vi "FlexMag - 23-03-2023.vi"() -> ()   [LabVIEW 2018] (continued)
        n7498 = feedback #256() -> (w13354:dbl)  [unwired: 1 in]
        n7499 = feedback-in #256(w13355) -> ()
        n7500 = feedback #257() -> (w13344:dbl)  [unwired: 1 in]
        n7501 = feedback-in #257(w13345) -> ()
        n7502 = feedback #258() -> (w13331:dbl)  [unwired: 1 in]
        n7503 = feedback-in #258(w13330) -> ()
        n7504 = feedback #259() -> (w13301:dbl)  [unwired: 1 in]
        n7505 = feedback-in #259(w13302) -> ()
        n7506 = feedback #260() -> (w13291:dbl)  [unwired: 1 in]
        n7507 = feedback-in #260(w13292) -> ()
        n7508 = feedback #261() -> (w13280:dbl)  [unwired: 1 in]
        n7509 = feedback-in #261(w13279) -> ()
        n7510 = feedback #262() -> (w13353:dbl)  [unwired: 1 in]
        n7511 = feedback-in #262(w13354) -> ()
        n7512 = feedback #263() -> (w13343:dbl)  [unwired: 1 in]
        n7513 = feedback-in #263(w13344) -> ()
        n7514 = feedback #264() -> (w13332:dbl)  [unwired: 1 in]
        n7515 = feedback-in #264(w13331) -> ()
        n7516 = feedback #265() -> (w13300:dbl)  [unwired: 1 in]
        n7517 = feedback-in #265(w13301) -> ()
        n7518 = feedback #266() -> (w13290:dbl)  [unwired: 1 in]
        n7519 = feedback-in #266(w13291) -> ()
        n7520 = feedback #267() -> (w13281:dbl)  [unwired: 1 in]
        n7521 = feedback-in #267(w13280) -> ()
        n7522 = feedback #268() -> (w13352:dbl)  [unwired: 1 in]
        n7523 = feedback-in #268(w13353) -> ()
        n7524 = feedback #269() -> (w13342:dbl)  [unwired: 1 in]
        n7525 = feedback-in #269(w13343) -> ()
        n7526 = feedback #270() -> (w13333:dbl)  [unwired: 1 in]
        n7527 = feedback-in #270(w13332) -> ()
        n7528 = feedback #271() -> (w13299:dbl)  [unwired: 1 in]
        n7529 = feedback-in #271(w13300) -> ()
        n7530 = feedback #272() -> (w13289:dbl)  [unwired: 1 in]
        n7531 = feedback-in #272(w13290) -> ()
        n7532 = feedback #273() -> (w13282:dbl)  [unwired: 1 in]
        n7533 = feedback-in #273(w13281) -> ()
        n7534 = feedback #274() -> (w13351:dbl)  [unwired: 1 in]
        n7535 = feedback-in #274(w13352) -> ()
        n7536 = feedback #275() -> (w13341:dbl)  [unwired: 1 in]
        n7537 = feedback-in #275(w13342) -> ()
        n7538 = feedback #276() -> (w13334:dbl)  [unwired: 1 in]
        n7539 = feedback-in #276(w13333) -> ()
        n7540 = feedback #277() -> (w13298:dbl)  [unwired: 1 in]
        n7541 = feedback-in #277(w13299) -> ()
        n7542 = feedback #278() -> (w13288:dbl)  [unwired: 1 in]
        n7543 = feedback-in #278(w13289) -> ()
        n7544 = feedback #279() -> (w13283:dbl)  [unwired: 1 in]
        n7545 = feedback-in #279(w13282) -> ()
        n7546 = feedback #280() -> (w13350:dbl)  [unwired: 1 in]
        n7547 = feedback-in #280(w13351) -> ()
        n7548 = feedback #281() -> (w13340:dbl)  [unwired: 1 in]
        n7549 = feedback-in #281(w13341) -> ()
        n7550 = feedback #282() -> (w13335:dbl)  [unwired: 1 in]
        n7551 = feedback-in #282(w13334) -> ()
        n7552 = feedback #283() -> (w13297:dbl)  [unwired: 1 in]
        n7553 = feedback-in #283(w13298) -> ()
        n7554 = feedback #284() -> (w13287:dbl)  [unwired: 1 in]
        n7555 = feedback-in #284(w13288) -> ()
        n7556 = feedback #285() -> (w13284:dbl)  [unwired: 1 in]
        n7557 = feedback-in #285(w13283) -> ()
        n7558 = feedback #286() -> (w13349:dbl)  [unwired: 1 in]
        n7559 = feedback-in #286(w13350) -> ()
        n7560 = feedback #287() -> (w13339:dbl)  [unwired: 1 in]
        n7561 = feedback-in #287(w13340) -> ()
        n7562 = feedback #288() -> (w13336:dbl)  [unwired: 1 in]
        n7563 = feedback-in #288(w13335) -> ()
        n7564 = feedback #289() -> (w13296:dbl)  [unwired: 1 in]
        n7565 = feedback-in #289(w13297) -> ()
        n7566 = feedback #290() -> (w13286:dbl)  [unwired: 1 in]
        n7567 = feedback-in #290(w13287) -> ()
        n7568 = feedback #291() -> (w13285:dbl)  [unwired: 1 in]
        n7569 = feedback-in #291(w13284) -> ()
        n7570 = feedback #292() -> (w13348:dbl)  [unwired: 1 in]
        n7571 = feedback-in #292(w13349) -> ()
        n7572 = feedback #293() -> (w13338:dbl)  [unwired: 1 in]
        n7573 = feedback-in #293(w13339) -> ()
        n7574 = feedback #294() -> (w13337:dbl)  [unwired: 1 in]
        n7575 = feedback-in #294(w13336) -> ()
        n7576 = Compound Arithmetic op=ADD(w13305, w13304, w13303, w13302, w13301, w13300, w13299, w13298, w13297, w13296) -> (w13308:dbl)
        n7577 = Compound Arithmetic op=ADD(w13295, w13294, w13293, w13292, w13291, w13290, w13289, w13288, w13287, w13286) -> (w13307:dbl)
        n7578 = Compound Arithmetic op=ADD(w13276, w13277, w13278, w13279, w13280, w13281, w13282, w13283, w13284, w13285) -> (w13306:dbl)
        n7579 = Compound Arithmetic op=ADD(w13357, w13356, w13355, w13354, w13353, w13352, w13351, w13350, w13349, w13348) -> (w13360:dbl)
        n7580 = Compound Arithmetic op=ADD(w13347, w13346, w13345, w13344, w13343, w13342, w13341, w13340, w13339, w13338) -> (w13359:dbl)
        n7581 = Compound Arithmetic op=ADD(w13328, w13329, w13330, w13331, w13332, w13333, w13334, w13335, w13336, w13337) -> (w13358:dbl)
        n7582 = Divide(x=w13308, y=10.0) -> (x/y=w13271:dbl)
        "ch4 cc ai(V)" <- w13271
        n7583 = Divide(x=w13360, y=10.0) -> (x/y=w13364:dbl)
        "ch3 cc ai(V)" <- w13364
        n7584 = Divide(x=w13307, y=10.0) -> (x/y=w13269:dbl)
        "ch4 pl pg ai(V)" <- w13269
        n7585 = Divide(x=w13306, y=10.0) -> (x/y=w13270:dbl)
        "ch4 ch pg ai(V)" <- w13270
        n7586 = Divide(x=w13359, y=10.0) -> (x/y=w13372:dbl)
        "ch3 pl pg ai(V)" <- w13372
        n7587 = Divide(x=w13358, y=10.0) -> (x/y=w13368:dbl)
        "ch3 ch pg ai(V)" <- w13368
        n7588 = Subtract(x=w13269, y=5.625) -> (x-y=w13268:dbl)
        n7589 = Subtract(x=w13270, y=5.625) -> (x-y=w13267:dbl)
        n7590 = Subtract(x=w13271, y=10.625) -> (x-y=w13261:dbl)
        n7591 = Subtract(x=w13372, y=5.625) -> (x-y=w13370:dbl)
        n7592 = Power Of 10(x=w13268) -> (10^x=w13266:dbl)
        n7593 = Subtract(x=w13368, y=5.625) -> (x-y=w13366:dbl)
        n7594 = Subtract(x=w13364, y=10.625) -> (x-y=w13362:dbl)
        n7595 = Power Of 10(x=w13261) -> (10^x=w13262:dbl)
        n7596 = Power Of 10(x=w13267) -> (10^x=w13264:dbl)
        n7597 = Power Of 10(x=w13370) -> (10^x=w13371:dbl)
        n7598 = Power Of 10(x=w13366) -> (10^x=w13365:dbl)
        n7599 = Power Of 10(x=w13362) -> (10^x=w13363:dbl)
        n7600 = In Range and Coerce(upper limit=1.0, x=w13262, lower limit=1e-09) -> (coerced(x)=w13260:dbl)  [unwired: 1 out]
        "ch4 cc torr" <- w13260
        n7601 = In Range and Coerce(upper limit=760.0, x=w13266, lower limit=0.000375) -> (coerced(x)=w13265:dbl)  [unwired: 1 out]
        "ch4 pl pg torr" <- w13265
        n7602 = In Range and Coerce(upper limit=760.0, x=w13371, lower limit=0.000375) -> (coerced(x)=w13369:dbl)  [unwired: 1 out]
        "ch3 pl pg  torr" <- w13369
        n7603 = In Range and Coerce(upper limit=760.0, x=w13264, lower limit=0.000375) -> (coerced(x)=w13263:dbl)  [unwired: 1 out]
        "ch4 ch pg torr" <- w13263
        n7604 = In Range and Coerce(upper limit=760.0, x=w13365, lower limit=0.000375) -> (coerced(x)=w13367:dbl)  [unwired: 1 out]
        "ch3 ch pg torr" <- w13367
        n7605 = In Range and Coerce(upper limit=1.0, x=w13363, lower limit=1e-09) -> (coerced(x)=w13361:dbl)  [unwired: 1 out]
        "ch3 cc torr" <- w13361
        n7606 = Multiply(x=w13260, y=1.33) -> (x*y=w13227:dbl)
        "ch4 cc mbar" <- w13227
        "ch4 cc mbar gui" <- w13227
        "ch4 cc mbar gui 1" <- w13227
        n7607 = Multiply(x=w13265, y=1.33) -> (x*y=w13229:dbl)
        "ch4 pl pg mbar" <- w13229
        "ch4 pl pg mbar gui" <- w13229
        "ch4 pl pg mbar gui 1" <- w13229
        n7608 = Multiply(x=w13369, y=1.33) -> (x*y=w13232:dbl)
        "ch3 pl pg mbar" <- w13232
        "ch3 pl pg mbar gui" <- w13232
        "ch3 pl pg mbar gui 1" <- w13232
        n7609 = Multiply(x=w13367, y=1.33) -> (x*y=w13231:dbl)
        "ch3 ch pg mbar" <- w13231
        "ch3 ch pg mbar gui" <- w13231
        "ch3 ch pg mbar gui 1" <- w13231
        n7610 = Multiply(x=w13361, y=1.33) -> (x*y=w13230:dbl)
        "ch3 cc mbar" <- w13230
        "ch3 cc mbar gui" <- w13230
        "ch3 cc mbar gui 1" <- w13230
        n7611 = Multiply(x=w13263, y=1.33) -> (x*y=w13228:dbl)
        "ch4 ch pg mbar" <- w13228
        "ch4 ch pg mbar gui" <- w13228
        "ch4 ch pg mbar gui 1" <- w13228
        n7612 = Number To Exponential String(number=w13231, precision (6)=i16 3) -> (E-format string=→"CH3 CH PG":string)  [unwired: 2 in]
        n7613 = Number To Exponential String(number=w13230, precision (6)=i16 3) -> (E-format string=→"CH3 CH CC":string)  [unwired: 2 in]
        n7614 = Number To Exponential String(number=w13232, precision (6)=i16 3) -> (E-format string=→"CH3 PL PG":string)  [unwired: 2 in]
        n7615 = Number To Exponential String(number=w13228, precision (6)=i16 3) -> (E-format string=→"CH4 CH PG":string)  [unwired: 2 in]
        n7616 = Number To Exponential String(number=w13227, precision (6)=i16 3) -> (E-format string=→"CH4 CH CC":string)  [unwired: 2 in]
        n7617 = Number To Exponential String(number=w13229, precision (6)=i16 3) -> (E-format string=→"CH4 PL PG":string)  [unwired: 2 in]
      }
    }
    n7618 = local read "MFC_Ar_Read_value"() -> (w12961:u16)
    n7619 = Wait Until Next ms Multiple(millisecond multiple=u32 300) -> ()  [unwired: 1 out]
    n7620 = Compound Arithmetic op=OR("ch1 ar set zero", "ch1 ar set zero auto") -> (w12986:bool)
    n7621 = Compound Arithmetic op=OR("ch4 ar set", "ch4 ar set auto") -> (w12990:bool)
    n7622 = Compound Arithmetic op=OR("ch4 ar set zero", "ch4 ar set zero auto") -> (w12989:bool)
    n7623 = Compound Arithmetic op=OR("ch1 ar set", "ch1 ar set auto") -> (w12983:bool)
    n7624 = Compound Arithmetic op=OR("ch2 ar set", "ch2 ar set auto") -> (w12994:bool)
    n7625 = Compound Arithmetic op=OR("ch2 ar set zero", "ch2 ar set zero auto") -> (w12995:bool)
    n7626 = Compound Arithmetic op=OR("ch3 ar set", "ch3 ar set auto") -> (w12997:bool)
    n7627 = Compound Arithmetic op=OR("ch3 ar set zero", "ch3 ar set zero auto") -> (w13005:bool)
    n7628 = Build Array(FALSE ("element"), w12983, w12986, w12994, w12995, w12997, w13005, w12990, w12989) -> (w12999:bool[])
    n7629 = Boolean Array To Number(Boolean array=w12999) -> (number=w13000:u32)
    n7630 = Less?(x=w12961, y=u16 20) -> (x < y?=w12964:bool)
    n7631 = Mantissa & Exponent(0:w13000) -> (2:w12998:dbl)  [unwired: 1 out]
    n7632 = case shown="False" w12964 {
      tunnel: [w13012 0] -> w12962
      tunnel: w12961 -> [w13012 _]
      frame False {
      }
      frame True {
      }
    }
    n7633 = local read "resolution"() -> (w12973:dbl)
    n7634 = Multiply(x=w12973, y=w12962) -> (x*y=w12972:dbl)
    n7635 = feedback-in #295(w12972) -> ()
    n7636 = feedback #295() -> (w12971:dbl)  [unwired: 1 in]
    n7637 = feedback #296() -> (w12970:dbl)  [unwired: 1 in]
    n7638 = feedback-in #296(w12971) -> ()
    n7639 = feedback #297() -> (w12969:dbl)  [unwired: 1 in]
    n7640 = feedback-in #297(w12970) -> ()
    n7641 = feedback #298() -> (w12968:dbl)  [unwired: 1 in]
    n7642 = feedback-in #298(w12969) -> ()
    n7643 = Compound Arithmetic op=ADD(w12972, w12971, w12970, w12969, w12968) -> (w12967:dbl)
    n7644 = Divide(x=w12967, y=5.0) -> (x/y=w12965:dbl)
    n7645 = case shown="0, Default" w12998 {
      tunnel: "ch3 mfc set safety" -> [_ _ _ _ _ w13058 _ _ _]
      tunnel: "ch3 argon mfc set" -> [_ _ _ _ _ w13057 _ _ _]
      tunnel: "ch1 argon mfc set" -> [_ w13033 _ _ _ _ _ _ _]
      tunnel: "ch1 mfc set safety" -> [_ w13034 _ _ _ _ _ _ _]
      tunnel: "ch2 argon mfc set" -> [_ _ _ w13046 _ _ _ _ _]
      tunnel: "ch2 mfc set safety" -> [_ _ _ w13045 _ _ _ _ _]
      tunnel: "ch4 mfc set safety" -> [_ _ _ _ _ _ _ w13070 _]
      tunnel: "ch4 argon mfc set" -> [_ _ _ _ _ _ _ w13069 _]
      tunnel: w12965 -> [w13015 _ _ _ _ _ _ _ _]
      frame 0, Default {
        n7646 = Multiply(x=w13015, y=40.0) -> (x*y=w13016:dbl)
        n7647 = local read "CH1_SoV_Ar_DI"() -> (w13023:bool)
        n7648 = local read "CH2_SoV_Ar_DI"() -> (w13022:bool)
        n7649 = local read "CH3_SoV_Ar_DI"() -> (w13021:bool)
        n7650 = local read "CH4_SoV_Ar_DI"() -> (w13020:bool)
        n7651 = case shown="True" w13023 {
          tunnel: [0.0 w13032] -> w13024
          tunnel: w13016 -> [_ w13032]
          frame False {
          }
          frame True {
          }
        }
        "ch1 argon mfc actual" <- w13024
        n7652 = case shown="True" w13022 {
          tunnel: [0.0 w13030] -> w13019
          tunnel: w13016 -> [_ w13030]
          frame False {
          }
          frame True {
          }
        }
        "ch2 argon mfc actual" <- w13019
        n7653 = case shown="True" w13021 {
          tunnel: [0.0 w13028] -> w13018
          tunnel: w13016 -> [_ w13028]
          frame False {
          }
          frame True {
          }
        }
        "ch3 argon mfc actual" <- w13018
        n7654 = case shown="True" w13020 {
          tunnel: [0.0 w13026] -> w13017
          tunnel: w13016 -> [_ w13026]
          frame False {
          }
          frame True {
          }
        }
        "ch4 argon mfc actual" <- w13017
      }
      frame 1 {
        # "ch1 ar set"
        n7655 = case shown="True" w13034 {
          tunnel: w13033 -> [_ w13036]
          frame False {
            n7656 = local write "Warning Message"("MFC cannot be setted on CH3" ("Warning Message")) -> ()
          }
          frame True {
            n7657 = flat-sequence {
              tunnel: w13036 -> [w13038]
              frame #0 {
                n7658 = local write "MFC_Ar_Set_value"(w13038) -> ()
                n7659 = Wait (ms)(milliseconds to wait=u32 500) -> ()  [unwired: 1 out]
              }
              frame #1 {
                n7660 = local write "MFC_Ar_Set"(TRUE ("MFC_Ar_Set")) -> ()
              }
            }
            n7661 = local write "ch1 ar set auto"(FALSE ("ch2 ar set auto")) -> ()
          }
        }
      }
      frame 2 {
        # "ch1 ar set zero"
        n7662 = flat-sequence {
          frame #0 {
            n7663 = local write "MFC_Ar_Set_value"(0.0 ("MFC_Ar_Set_value")) -> ()
            n7664 = Wait (ms)(milliseconds to wait=u32 500) -> ()  [unwired: 1 out]
          }
          frame #1 {
            n7665 = local write "MFC_Ar_Set"(TRUE ("MFC_Ar_Set")) -> ()
          }
        }
        n7666 = local write "ch1 ar set zero auto"(FALSE ("ch2 ar set auto")) -> ()
      }
      frame 3 {
        # "ch2 ar set"
        n7667 = case shown="True" w13045 {
          tunnel: w13046 -> [_ w13048]
          frame False {
            n7668 = local write "Warning Message"("MFC cannot be setted on CH2" ("Warning Message")) -> ()
          }
          frame True {
            n7669 = flat-sequence {
              tunnel: w13048 -> [w13050]
              frame #0 {
                n7670 = local write "MFC_Ar_Set_value"(w13050) -> ()
                n7671 = Wait (ms)(milliseconds to wait=u32 500) -> ()  [unwired: 1 out]
              }
              frame #1 {
                n7672 = local write "MFC_Ar_Set"(TRUE ("MFC_Ar_Set")) -> ()
              }
            }
            n7673 = local write "ch2 ar set auto"(FALSE ("ch2 ar set auto")) -> ()
          }
        }
      }
      frame 4 {
        # "ch2 ar set zero"
        n7674 = flat-sequence {
          frame #0 {
            n7675 = local write "MFC_Ar_Set_value"(0.0 ("MFC_Ar_Set_value")) -> ()
            n7676 = Wait (ms)(milliseconds to wait=u32 500) -> ()  [unwired: 1 out]
          }
          frame #1 {
            n7677 = local write "MFC_Ar_Set"(TRUE ("MFC_Ar_Set")) -> ()
          }
        }
        n7678 = local write "ch2 ar set zero auto"(FALSE ("ch2 ar set auto")) -> ()
      }
      frame 5 {
        # "ch3 ar set"
        n7679 = case shown="True" w13058 {
          tunnel: w13057 -> [_ w13060]
          frame False {
            n7680 = local write "Warning Message"("MFC cannot be setted on CH3" ("Warning Message")) -> ()
          }
          frame True {
            n7681 = flat-sequence {
              tunnel: w13060 -> [w13062]
              frame #0 {
                n7682 = local write "MFC_Ar_Set_value"(w13062) -> ()
                n7683 = Wait (ms)(milliseconds to wait=u32 500) -> ()  [unwired: 1 out]
              }
              frame #1 {
                n7684 = local write "MFC_Ar_Set"(TRUE ("MFC_Ar_Set")) -> ()
              }
            }
            n7685 = local write "ch3 ar set auto"(FALSE ("ch2 ar set auto")) -> ()
          }
        }
      }
      frame 6 {
        # "ch3 ar set zero"
        n7686 = flat-sequence {
          frame #0 {
            n7687 = local write "MFC_Ar_Set_value"(0.0 ("MFC_Ar_Set_value")) -> ()
            n7688 = Wait (ms)(milliseconds to wait=u32 500) -> ()  [unwired: 1 out]
          }
          frame #1 {
            n7689 = local write "MFC_Ar_Set"(TRUE ("MFC_Ar_Set")) -> ()
          }
        }
        n7690 = local write "ch3 ar set zero auto"(FALSE ("ch2 ar set auto")) -> ()
      }
      frame 7 {
        # "ch4 ar set"
        n7691 = case shown="True" w13070 {
          tunnel: w13069 -> [_ w13072]
          frame False {
            n7692 = local write "Warning Message"("MFC cannot be setted on CH3" ("Warning Message")) -> ()
          }
          frame True {
            n7693 = flat-sequence {
              tunnel: w13072 -> [w13074]
              frame #0 {
                n7694 = local write "MFC_Ar_Set_value"(w13074) -> ()
                n7695 = Wait (ms)(milliseconds to wait=u32 500) -> ()  [unwired: 1 out]
              }
              frame #1 {
                n7696 = local write "MFC_Ar_Set"(TRUE ("MFC_Ar_Set")) -> ()
              }
            }
            n7697 = local write "ch4 ar set auto"(FALSE ("ch2 ar set auto")) -> ()
          }
        }
      }
      frame 8 {
        # "ch4 ar set zero"
        n7698 = flat-sequence {
          frame #0 {
            n7699 = local write "MFC_Ar_Set_value"(0.0 ("MFC_Ar_Set_value")) -> ()
            n7700 = Wait (ms)(milliseconds to wait=u32 500) -> ()  [unwired: 1 out]
          }
          frame #1 {
            n7701 = local write "MFC_Ar_Set"(TRUE ("MFC_Ar_Set")) -> ()
          }
        }
        n7702 = local write "ch4 ar set zero auto"(FALSE ("ch2 ar set auto")) -> ()
      }
    }
  }
  n7703 = VISA Close(VISA resource name=w28, error in (no error)=w29) -> ()  [unwired: 1 out]
  n7704 = VISA Close(VISA resource name=w22, error in (no error)=w23) -> ()  [unwired: 1 out]
  n7705 = VISA Close(VISA resource name=w72, error in (no error)=w73) -> ()  [unwired: 1 out]
  n7706 = while {
    stop <- FALSE stop-if-true
    n7707 = Wait Until Next ms Multiple(millisecond multiple=u32 300) -> ()  [unwired: 1 out]
    n7708 = stacked-sequence {
      frame #0 {
        n7709 = feedback #299() -> (w13377:bool)  [unwired: 1 in]
        n7710 = feedback #300() -> (w13383:bool)  [unwired: 1 in]
        n7711 = feedback #301() -> (w13379:bool)  [unwired: 1 in]
        n7712 = feedback #302() -> (w13386:bool)  [unwired: 1 in]
        n7713 = case shown="True" "ch4 pumpdown error" {
          tunnel: w13377 -> [_ w13396]
          tunnel: [TRUE FALSE] -> w13376
          frame False {
          }
          frame True {
            n7714 = call "Elapsed Time60"("Auto Reset"=w13396) -> ("Elapsed Time (s)"=w13388:dbl)  [unwired: 11 in, 7 out]
            n7715 = In Range and Coerce(upper limit=1.5, x=w13388, lower limit=0.0) -> (In Range?=w13392:bool)  [unwired: 1 out]
            n7716 = In Range and Coerce(upper limit=9.0, x=w13388, lower limit=7.5) -> (In Range?=w13389:bool)  [unwired: 1 out]
            n7717 = case shown="True" w13392 {
              frame False {
              }
              frame True {
                w13399 = FALSE ("CH1_CC_DO")
                w13400 = TRUE ("Buzzer DO")
                n7718 = local write "Buzzer DO"(w13400) -> ()
                n7719 = local write "Tp4 auto stop"(w13400) -> ()
                n7720 = local write "pcgv4 auto close"(w13400) -> ()
                n7721 = local write "System Status"("CH4 PUMPDOWN ERROR" ("System Status")) -> ()
                n7722 = local write "CH4_CC_DO"(w13399) -> ()
                n7723 = local write "ch4 pumpdown alg"(w13399) -> ()
                n7724 = local write "Pump Down CH4"(w13399) -> ()
              }
            }
            n7725 = case shown="True" w13389 {
              frame False {
              }
              frame True {
                w13397 = FALSE ("Buzzer DO")
                n7726 = local write "Buzzer DO"(w13397) -> ()
                n7727 = local write "ch4 pumpdown error"(w13397) -> ()
                n7728 = local write "System Status"("SEMI-AUTOMATIC MODE" ("System Status")) -> ()
              }
            }
          }
        }
        n7729 = feedback-in #299(w13376) -> ()
        n7730 = case shown="True" "ch2 pumpdown error" {
          tunnel: w13383 -> [_ w13426]
          tunnel: [TRUE FALSE] -> w13382
          frame False {
          }
          frame True {
            n7731 = call "Elapsed Time58"("Auto Reset"=w13426) -> ("Elapsed Time (s)"=w13418:dbl)  [unwired: 11 in, 7 out]
            n7732 = In Range and Coerce(upper limit=1.5, x=w13418, lower limit=0.0) -> (In Range?=w13422:bool)  [unwired: 1 out]
            n7733 = In Range and Coerce(upper limit=9.0, x=w13418, lower limit=7.5) -> (In Range?=w13419:bool)  [unwired: 1 out]
            n7734 = case shown="True" w13422 {
              frame False {
              }
              frame True {
                w13429 = FALSE ("CH1_CC_DO")
                w13430 = TRUE ("Buzzer DO")
                n7735 = local write "Buzzer DO"(w13430) -> ()
                n7736 = local write "Tp2 auto stop"(w13430) -> ()
                n7737 = local write "pcgv2 auto close"(w13430) -> ()
                n7738 = local write "System Status"("CH2 PUMPDOWN ERROR" ("System Status")) -> ()
                n7739 = local write "CH2_CC_DO"(w13429) -> ()
                n7740 = local write "ch2 pumpdown alg"(w13429) -> ()
                n7741 = local write "Pump Down CH2"(w13429) -> ()
              }
            }
            n7742 = case shown="True" w13419 {
              frame False {
              }
              frame True {
                w13427 = FALSE ("Buzzer DO")
                n7743 = local write "Buzzer DO"(w13427) -> ()
                n7744 = local write "ch2 pumpdown error"(w13427) -> ()
                n7745 = local write "System Status"("SEMI-AUTOMATIC MODE" ("System Status")) -> ()
              }
            }
          }
        }
        n7746 = feedback-in #300(w13382) -> ()
        n7747 = case shown="True" "ch3 pumpdown error" {
          tunnel: w13379 -> [_ w13411]
          tunnel: [TRUE FALSE] -> w13380
          frame False {
          }
          frame True {
            n7748 = call "Elapsed Time59"("Auto Reset"=w13411) -> ("Elapsed Time (s)"=w13403:dbl)  [unwired: 11 in, 7 out]
            n7749 = In Range and Coerce(upper limit=1.5, x=w13403, lower limit=0.0) -> (In Range?=w13407:bool)  [unwired: 1 out]
            n7750 = In Range and Coerce(upper limit=9.0, x=w13403, lower limit=7.5) -> (In Range?=w13404:bool)  [unwired: 1 out]
            n7751 = case shown="True" w13407 {
              frame False {
              }
              frame True {
                w13414 = FALSE ("CH1_CC_DO")
                w13415 = TRUE ("Buzzer DO")
                n7752 = local write "Buzzer DO"(w13415) -> ()
                n7753 = local write "Tp3 auto stop"(w13415) -> ()
                n7754 = local write "pcgv3 auto close"(w13415) -> ()
                n7755 = local write "System Status"("CH3 PUMPDOWN ERROR" ("System Status")) -> ()
                n7756 = local write "CH3_CC_DO"(w13414) -> ()
                n7757 = local write "ch3 pumpdown alg"(w13414) -> ()
                n7758 = local write "Pump Down CH3"(w13414) -> ()
              }
            }
            n7759 = case shown="True" w13404 {
              frame False {
              }
              frame True {
                w13412 = FALSE ("Buzzer DO")
                n7760 = local write "Buzzer DO"(w13412) -> ()
                n7761 = local write "ch3 pumpdown error"(w13412) -> ()
                n7762 = local write "System Status"("SEMI-AUTOMATIC MODE" ("System Status")) -> ()
              }
            }
          }
        }
        n7763 = feedback-in #301(w13380) -> ()
        n7764 = case shown="True" "ch1 pumpdown error" {
          tunnel: w13386 -> [_ w13441]
          tunnel: [TRUE FALSE] -> w13385
          frame False {
          }
          frame True {
            n7765 = call "Elapsed Time48"("Auto Reset"=w13441) -> ("Elapsed Time (s)"=w13433:dbl)  [unwired: 11 in, 7 out]
            n7766 = In Range and Coerce(upper limit=1.5, x=w13433, lower limit=0.0) -> (In Range?=w13437:bool)  [unwired: 1 out]
            n7767 = In Range and Coerce(upper limit=9.0, x=w13433, lower limit=7.5) -> (In Range?=w13434:bool)  [unwired: 1 out]
            n7768 = case shown="True" w13437 {
              frame False {
              }
              frame True {
                w13444 = FALSE ("CH1_CC_DO")
                w13445 = TRUE ("Buzzer DO")
                n7769 = local write "Buzzer DO"(w13445) -> ()
                n7770 = local write "Tp1 auto stop"(w13445) -> ()
                n7771 = local write "pcgv1 auto close"(w13445) -> ()
                n7772 = local write "System Status"("CH1 PUMPDOWN ERROR" ("System Status")) -> ()
                n7773 = local write "CH1_CC_DO"(w13444) -> ()
                n7774 = local write "ch1 pumpdown alg"(w13444) -> ()
                n7775 = local write "Pump Down CH1"(w13444) -> ()
              }
            }
            n7776 = case shown="True" w13434 {
              frame False {
              }
              frame True {
                w13442 = FALSE ("Buzzer DO")
                n7777 = local write "Buzzer DO"(w13442) -> ()
                n7778 = local write "ch1 pumpdown error"(w13442) -> ()
                n7779 = local write "System Status"("SEMI-AUTOMATIC MODE" ("System Status")) -> ()
              }
            }
          }
        }
        n7780 = feedback-in #302(w13385) -> ()
      }
      frame #1 {
        n7781 = feedback #303() -> (w13449:bool)  [unwired: 1 in]
        n7782 = feedback #304() -> (w13452:bool)  [unwired: 1 in]
        n7783 = feedback #305() -> (w13458:bool)  [unwired: 1 in]
        n7784 = feedback #306() -> (w13454:bool)  [unwired: 1 in]
        n7785 = case shown="True" "ch4 shutdown error" {
          tunnel: w13449 -> [_ w13468]
          tunnel: [TRUE FALSE] -> w13450
          frame False {
          }
          frame True {
            n7786 = call "Elapsed Time64"("Auto Reset"=w13468) -> ("Elapsed Time (s)"=w13460:dbl)  [unwired: 11 in, 7 out]
            n7787 = In Range and Coerce(upper limit=1.5, x=w13460, lower limit=0.0) -> (In Range?=w13464:bool)  [unwired: 1 out]
            n7788 = In Range and Coerce(upper limit=9.0, x=w13460, lower limit=7.5) -> (In Range?=w13461:bool)  [unwired: 1 out]
            n7789 = case shown="True" w13464 {
              frame False {
              }
              frame True {
                w13471 = FALSE ("CH1_CC_DO")
                w13472 = TRUE ("Buzzer DO")
                n7790 = local write "Buzzer DO"(w13472) -> ()
                n7791 = local write "Tp4 auto stop"(w13472) -> ()
                n7792 = local write "pcgv4 auto close"(w13472) -> ()
                n7793 = local write "System Status"("CH4 SHUTDOWN ERROR" ("System Status")) -> ()
                n7794 = local write "CH4_CC_DO"(w13471) -> ()
                n7795 = local write "ch4 shutdown alg"(w13471) -> ()
                n7796 = local write "Shut Down CH4"(w13471) -> ()
              }
            }
            n7797 = case shown="True" w13461 {
              frame False {
              }
              frame True {
                w13469 = FALSE ("Buzzer DO")
                n7798 = local write "Buzzer DO"(w13469) -> ()
                n7799 = local write "ch4 shutdown error"(w13469) -> ()
                n7800 = local write "System Status"("SEMI-AUTOMATIC MODE" ("System Status")) -> ()
              }
            }
          }
        }
        n7801 = feedback-in #303(w13450) -> ()
        n7802 = case shown="True" "ch3 shutdown error" {
          tunnel: w13452 -> [_ w13483]
          tunnel: [TRUE FALSE] -> w13451
          frame False {
          }
          frame True {
            n7803 = call "Elapsed Time63"("Auto Reset"=w13483) -> ("Elapsed Time (s)"=w13475:dbl)  [unwired: 11 in, 7 out]
            n7804 = In Range and Coerce(upper limit=1.5, x=w13475, lower limit=0.0) -> (In Range?=w13479:bool)  [unwired: 1 out]
            n7805 = In Range and Coerce(upper limit=9.0, x=w13475, lower limit=7.5) -> (In Range?=w13476:bool)  [unwired: 1 out]
            n7806 = case shown="True" w13479 {
              frame False {
              }
              frame True {
                w13486 = FALSE ("CH1_CC_DO")
                w13487 = TRUE ("Buzzer DO")
                n7807 = local write "Buzzer DO"(w13487) -> ()
                n7808 = local write "Tp3 auto stop"(w13487) -> ()
                n7809 = local write "pcgv3 auto close"(w13487) -> ()
                n7810 = local write "System Status"("CH3 SHUTDOWN ERROR" ("System Status")) -> ()
                n7811 = local write "CH3_CC_DO"(w13486) -> ()
                n7812 = local write "ch3 shutdown alg"(w13486) -> ()
                n7813 = local write "Shut Down CH3"(w13486) -> ()
              }
            }
            n7814 = case shown="True" w13476 {
              frame False {
              }
              frame True {
                w13484 = FALSE ("Buzzer DO")
                n7815 = local write "Buzzer DO"(w13484) -> ()
                n7816 = local write "ch3 shutdown error"(w13484) -> ()
                n7817 = local write "System Status"("SEMI-AUTOMATIC MODE" ("System Status")) -> ()
              }
            }
          }
        }
        n7818 = feedback-in #304(w13451) -> ()
        n7819 = case shown="True" "ch1 shutdown error" {
          tunnel: w13458 -> [_ w13513]
          tunnel: [TRUE FALSE] -> w13457
          frame False {
          }
          frame True {
            n7820 = call "Elapsed Time61"("Auto Reset"=w13513) -> ("Elapsed Time (s)"=w13505:dbl)  [unwired: 11 in, 7 out]
            n7821 = In Range and Coerce(upper limit=1.5, x=w13505, lower limit=0.0) -> (In Range?=w13509:bool)  [unwired: 1 out]
            n7822 = In Range and Coerce(upper limit=9.0, x=w13505, lower limit=7.5) -> (In Range?=w13506:bool)  [unwired: 1 out]
            n7823 = case shown="True" w13509 {
              frame False {
              }
              frame True {
                w13516 = FALSE ("CH1_CC_DO")
                w13517 = TRUE ("Buzzer DO")
                n7824 = local write "Buzzer DO"(w13517) -> ()
                n7825 = local write "Tp1 auto stop"(w13517) -> ()
                n7826 = local write "pcgv1 auto close"(w13517) -> ()
                n7827 = local write "System Status"("CH1 SHUTDOWN ERROR" ("System Status")) -> ()
                n7828 = local write "CH1_CC_DO"(w13516) -> ()
                n7829 = local write "ch2 shutdown alg"(w13516) -> ()
                n7830 = local write "Shut Down CH1"(w13516) -> ()
              }
            }
            n7831 = case shown="True" w13506 {
              frame False {
              }
              frame True {
                w13514 = FALSE ("Buzzer DO")
                n7832 = local write "ch1 shutdown error"(w13514) -> ()
                n7833 = local write "Buzzer DO"(w13514) -> ()
                n7834 = local write "System Status"("SEMI-AUTOMATIC MODE" ("System Status")) -> ()
              }
            }
          }
        }
        n7835 = feedback-in #305(w13457) -> ()
        n7836 = case shown="True" "ch2 shutdown error" {
          tunnel: w13454 -> [_ w13498]
          tunnel: [TRUE FALSE] -> w13455
          frame False {
          }
          frame True {
            n7837 = call "Elapsed Time62"("Auto Reset"=w13498) -> ("Elapsed Time (s)"=w13490:dbl)  [unwired: 11 in, 7 out]
            n7838 = In Range and Coerce(upper limit=1.5, x=w13490, lower limit=0.0) -> (In Range?=w13494:bool)  [unwired: 1 out]
            n7839 = In Range and Coerce(upper limit=9.0, x=w13490, lower limit=7.5) -> (In Range?=w13491:bool)  [unwired: 1 out]
            n7840 = case shown="True" w13494 {
              frame False {
              }
              frame True {
                w13501 = FALSE ("CH1_CC_DO")
                w13502 = TRUE ("Buzzer DO")
                n7841 = local write "Buzzer DO"(w13502) -> ()
                n7842 = local write "Tp2 auto stop"(w13502) -> ()
                n7843 = local write "pcgv2 auto close"(w13502) -> ()
                n7844 = local write "System Status"("CH2 SHUTDOWN ERROR" ("System Status")) -> ()
                n7845 = local write "CH2_CC_DO"(w13501) -> ()
                n7846 = local write "ch2 shutdown alg"(w13501) -> ()
                n7847 = local write "Shut Down CH2"(w13501) -> ()
              }
            }
            n7848 = case shown="True" w13491 {
              frame False {
              }
              frame True {
                w13499 = FALSE ("Buzzer DO")
                n7849 = local write "Buzzer DO"(w13499) -> ()
                n7850 = local write "ch2 shutdown error"(w13499) -> ()
                n7851 = local write "System Status"("SEMI-AUTOMATIC MODE" ("System Status")) -> ()
              }
            }
          }
        }
        n7852 = feedback-in #306(w13455) -> ()
      }
      frame #2 {
        n7853 = feedback #307() -> (w13523:bool)  [unwired: 1 in]
        n7854 = feedback #308() -> (w13520:bool)  [unwired: 1 in]
        n7855 = feedback #309() -> (w13527:bool)  [unwired: 1 in]
        n7856 = case shown="True" "roll error" {
          tunnel: [TRUE FALSE] -> w13524
          tunnel: w13523 -> [_ w13550]
          frame False {
          }
          frame True {
            n7857 = call "Elapsed Time139"("Auto Reset"=w13550) -> ("Elapsed Time (s)"=w13543:dbl)  [unwired: 11 in, 7 out]
            n7858 = local read "coating start"() -> (w13542:bool)
            n7859 = In Range and Coerce(upper limit=5.0, x=w13543, lower limit=0.0) -> (In Range?=w13547:bool)  [unwired: 1 out]
            n7860 = In Range and Coerce(upper limit=7.0, x=w13543, lower limit=5.5) -> (In Range?=w13544:bool)  [unwired: 1 out]
            n7861 = case shown="True" w13547 {
              frame False {
              }
              frame True {
                w13558 = FALSE
                w13557 = FALSE
                n7862 = local write "CH1_Motor DO"(w13557) -> ()
                n7863 = local write "CH2_Motor DO"(w13557) -> ()
                n7864 = local write "CH3_Motor DO"(w13557) -> ()
                n7865 = local write "CH4_Motor DO"(w13557) -> ()
                n7866 = local write "System Status"("Rolling Error" ("System Status")) -> ()
                n7867 = local write "forward roll"(w13558) -> ()
                n7868 = local write "back roll"(w13558) -> ()
                n7869 = local write "position"(w13558) -> ()
                n7870 = local write "cycle roll start"(FALSE) -> ()
                n7871 = local write "Buzzer DO"(TRUE ("Buzzer DO")) -> ()
              }
            }
            n7872 = case shown="True" w13544 {
              frame False {
              }
              frame True {
                n7873 = local write "Buzzer DO"(FALSE ("Buzzer DO")) -> ()
                n7874 = local write "System Status"("SEMI-AUTOMATIC MODE" ("System Status")) -> ()
                n7875 = local write "roll error"(FALSE) -> ()
              }
            }
            n7876 = case shown="True" w13542 {
              frame False {
              }
              frame True {
                n7877 = local write "coating error"(TRUE ("coating error")) -> ()
              }
            }
          }
        }
        n7878 = feedback-in #307(w13524) -> ()
        n7879 = case shown="True" "trns error" {
          tunnel: w13527 -> [_ w13574]
          tunnel: [TRUE FALSE] -> w13526
          frame False {
          }
          frame True {
            n7880 = local read "coating start"() -> (w13562:bool)
            n7881 = call "Elapsed Time138"("Auto Reset"=w13574) -> ("Elapsed Time (s)"=w13564:dbl)  [unwired: 11 in, 7 out]
            n7882 = case shown="True" w13562 {
              frame False {
              }
              frame True {
                n7883 = local write "coating error"(TRUE ("coating error")) -> ()
              }
            }
            n7884 = flat-sequence {
              frame #0 {
                n7885 = local write "Cassette_Servo_Speed AO"(0.0 ("Cassette_Servo_Speed AO")) -> ()
              }
              frame #1 {
                n7886 = local write "Cassette_Servo_Speed Set"(TRUE ("Cassette_Servo_Speed Set")) -> ()
              }
            }
            n7887 = In Range and Coerce(upper limit=11.5, x=w13564, lower limit=10.0) -> (In Range?=w13567:bool)  [unwired: 1 out]
            n7888 = In Range and Coerce(upper limit=9.5, x=w13564, lower limit=0.0) -> (In Range?=w13570:bool)  [unwired: 1 out]
            n7889 = In Range and Coerce(upper limit=1.0, x=w13564, lower limit=0.0) -> (In Range?=w13563:bool)  [unwired: 1 out]
            n7890 = case shown="True" w13570 {
              frame False {
              }
              frame True {
                w13585 = FALSE
                w13586 = FALSE
                w13587 = FALSE
                n7891 = local write "ch1-2 transfer"(w13586) -> ()
                n7892 = local write "ch2-3 transfer"(w13586) -> ()
                n7893 = local write "ch3-4 transfer"(w13586) -> ()
                n7894 = local write "ch2-1 transfer"(w13586) -> ()
                n7895 = local write "ch3-2 transfer"(w13586) -> ()
                n7896 = local write "ch4-3 transfer"(w13586) -> ()
                n7897 = local write "1-2 tr"(w13587) -> ()
                n7898 = local write "1-3 tr"(w13587) -> ()
                n7899 = local write "1-4 tr"(w13587) -> ()
                n7900 = local write "2-1 tr"(w13587) -> ()
                n7901 = local write "2-3 tr"(w13587) -> ()
                n7902 = local write "2-4 tr"(w13587) -> ()
                n7903 = local write "3-1 tr"(w13587) -> ()
                n7904 = local write "3-2 tr"(w13587) -> ()
                n7905 = local write "3-4 tr"(w13587) -> ()
                n7906 = local write "4-1 tr"(w13587) -> ()
                n7907 = local write "4-2 tr"(w13587) -> ()
                n7908 = local write "4-3 tr"(w13587) -> ()
                n7909 = local write "Casette_Servo_Start/Stop DO"(FALSE ("Casette_Servo_Start/Stop DO")) -> ()
                n7910 = local write "transfer atm"(w13585) -> ()
                n7911 = local write "transfer atm auto"(w13585) -> ()
                n7912 = local write "transfer vacuum"(w13585) -> ()
                n7913 = local write "transfer vacuum auto"(w13585) -> ()
                n7914 = local write "TRNS atm alg"(w13585) -> ()
                n7915 = local write "TRNS vacuum alg"(w13585) -> ()
                n7916 = local write "trns pre check"(w13585) -> ()
                n7917 = local write "coating start"(FALSE) -> ()
                n7918 = local write "trns V?"(FALSE) -> ()
                n7919 = local write "System Status"("Transfer Error" ("System Status")) -> ()
              }
            }
            n7920 = case shown="True" w13567 {
              frame False {
              }
              frame True {
                w13580 = FALSE ("Buzzer DO")
                n7921 = local write "Buzzer DO"(w13580) -> ()
                n7922 = local write "trns error"(w13580) -> ()
                n7923 = local write "System Status"("SEMI-AUTOMATIC MODE" ("System Status")) -> ()
                n7924 = local write "coating start"(FALSE) -> ()
              }
            }
            n7925 = case shown="True" w13563 {
              frame False {
              }
              frame True {
                n7926 = local write "Buzzer DO"(TRUE ("Buzzer DO")) -> ()
              }
            }
          }
        }
        n7927 = feedback-in #309(w13526) -> ()
        n7928 = case shown="True" "ABORT" {
          tunnel: w13520 -> [_ w13537]
          tunnel: [TRUE FALSE] -> w13519
          frame False {
          }
          frame True {
            w13538 = TRUE
            n7929 = local write "abort ch1"(w13538) -> ()
            n7930 = local write "abort ch2"(w13538) -> ()
            n7931 = local write "abort ch3"(w13538) -> ()
            n7932 = local write "abort ch4"(w13538) -> ()
            n7933 = call "Elapsed Time154"("Auto Reset"=w13537) -> ("Elapsed Time (s)"=w13531:dbl)  [unwired: 11 in, 7 out]
            n7934 = In Range and Coerce(upper limit=7.0, x=w13531, lower limit=5.5) -> (In Range?=w13530:bool)  [unwired: 1 out]
            n7935 = In Range and Coerce(upper limit=5.0, x=w13531, lower limit=0.0) -> (In Range?=w13529:bool)  [unwired: 1 out]
            n7936 = case shown="True" w13529 {
              frame False {
              }
              frame True {
                n7937 = local write "System Status"("SYSTEM ABORTED !" ("System Status")) -> ()
              }
            }
            n7938 = case shown="True" w13530 {
              frame False {
              }
              frame True {
                n7939 = local write "ABORT"(FALSE ("ABORT")) -> ()
              }
            }
          }
        }
        n7940 = feedback-in #308(w13519) -> ()
      }
      frame #3 {
        # "argon \nflow off"
        n7941 = feedback #310() -> (w13594:bool)  [unwired: 1 in]
        n7942 = feedback #311() -> (w13590:bool)  [unwired: 1 in]
        n7943 = case shown="True" "abort ch1" {
          tunnel: w13594 -> [_ w13647]
          tunnel: [TRUE FALSE] -> w13592
          frame False {
          }
          frame True {
            n7944 = call "Elapsed Time150"("Auto Reset"=w13647) -> ("Elapsed Time (s)"=w13631:dbl)  [unwired: 11 in, 7 out]
            n7945 = In Range and Coerce(upper limit=5.5, x=w13631, lower limit=0.0) -> (In Range?=w13643:bool)  [unwired: 1 out]
            n7946 = In Range and Coerce(upper limit=1.5, x=w13631, lower limit=0.0) -> (In Range?=w13637:bool)  [unwired: 1 out]
            n7947 = In Range and Coerce(upper limit=9.5, x=w13631, lower limit=8.5) -> (In Range?=w13640:bool)  [unwired: 1 out]
            n7948 = In Range and Coerce(upper limit=8.0, x=w13631, lower limit=7.0) -> (In Range?=w13630:bool)  [unwired: 1 out]
            n7949 = In Range and Coerce(upper limit=6.5, x=w13631, lower limit=5.5) -> (In Range?=w13634:bool)  [unwired: 1 out]
            n7950 = case shown="True" w13640 {
              frame False {
              }
              frame True {
                n7951 = local write "Buzzer DO"(FALSE ("Buzzer DO")) -> ()
                n7952 = local write "System Status"("SEMI-AUTOMATIC MODE" ("System Status")) -> ()
                n7953 = local write "abort ch1"(FALSE ("Buzzer DO")) -> ()
              }
            }
            n7954 = case shown="True" w13634 {
              frame False {
              }
              frame True {
                n7955 = local write "CH1_TP_BV_DO"(FALSE ("Buzzer DO")) -> ()
              }
            }
            n7956 = case shown="True" w13643 {
              frame False {
              }
              frame True {
                w13658 = FALSE
                w13659 = FALSE
                w13656 = FALSE ("CH1_CC_DO")
                n7957 = local write "Buzzer DO"(TRUE ("Buzzer DO")) -> ()
                n7958 = local write "1-2 tr"(w13659) -> ()
                n7959 = local write "1-3 tr"(w13659) -> ()
                n7960 = local write "1-4 tr"(w13659) -> ()
                n7961 = local write "2-1 tr"(w13659) -> ()
                n7962 = local write "2-3 tr"(w13659) -> ()
                n7963 = local write "2-4 tr"(w13659) -> ()
                n7964 = local write "3-1 tr"(w13659) -> ()
                n7965 = local write "3-2 tr"(w13659) -> ()
                n7966 = local write "3-4 tr"(w13659) -> ()
                n7967 = local write "4-1 tr"(w13659) -> ()
                n7968 = local write "4-2 tr"(w13659) -> ()
                n7969 = local write "4-3 tr"(w13659) -> ()
                n7970 = local write "Casette_Servo_Start/Stop DO"(FALSE ("Casette_Servo_Start/Stop DO")) -> ()
                n7971 = local write "CH1_Trns_BP_Left_DO"(FALSE ("CH1_Trns_BP_Left_DO")) -> ()
                n7972 = local write "CH1_CC_DO"(w13656) -> ()
                n7973 = local write "ch1 pumpdown alg"(w13656) -> ()
                n7974 = local write "Pump Down CH1"(w13656) -> ()
                n7975 = local write "ch1 shutdown alg"(w13656) -> ()
                n7976 = local write "Shut Down CH1"(w13656) -> ()
                n7977 = local write "ch1-2 transfer"(w13658) -> ()
                n7978 = local write "ch2-3 transfer"(w13658) -> ()
                n7979 = local write "ch3-4 transfer"(w13658) -> ()
                n7980 = local write "ch2-1 transfer"(w13658) -> ()
                n7981 = local write "ch3-2 transfer"(w13658) -> ()
                n7982 = local write "ch4-3 transfer"(w13658) -> ()
              }
            }
            n7983 = case shown="True" w13637 {
              frame False {
              }
              frame True {
                w13652 = TRUE ("Buzzer DO")
                n7984 = local write "Tp1 auto stop"(w13652) -> ()
                n7985 = local write "pcgv1 auto close"(w13652) -> ()
                n7986 = local write "System Status"("CH1 ABORTED" ("System Status")) -> ()
              }
            }
            n7987 = case shown="True" w13630 {
              frame False {
              }
              frame True {
                n7988 = local write "CH1_PL_VBV_DO"(TRUE) -> ()
                n7989 = local write "CH1_MP_DO"(FALSE ("Buzzer DO")) -> ()
              }
            }
          }
        }
        n7990 = feedback-in #310(w13592) -> ()
        n7991 = case shown="True" "abort ch2" {
          tunnel: w13590 -> [_ w13613]
          tunnel: [TRUE FALSE] -> w13591
          frame False {
          }
          frame True {
            n7992 = call "Elapsed Time151"("Auto Reset"=w13613) -> ("Elapsed Time (s)"=w13597:dbl)  [unwired: 11 in, 7 out]
            n7993 = In Range and Coerce(upper limit=5.5, x=w13597, lower limit=0.0) -> (In Range?=w13609:bool)  [unwired: 1 out]
            n7994 = In Range and Coerce(upper limit=1.5, x=w13597, lower limit=0.0) -> (In Range?=w13603:bool)  [unwired: 1 out]
            n7995 = In Range and Coerce(upper limit=9.5, x=w13597, lower limit=8.5) -> (In Range?=w13606:bool)  [unwired: 1 out]
            n7996 = In Range and Coerce(upper limit=8.0, x=w13597, lower limit=7.0) -> (In Range?=w13596:bool)  [unwired: 1 out]
            n7997 = In Range and Coerce(upper limit=6.5, x=w13597, lower limit=5.5) -> (In Range?=w13600:bool)  [unwired: 1 out]
            n7998 = case shown="True" w13606 {
              frame False {
              }
              frame True {
                n7999 = local write "Buzzer DO"(FALSE ("Buzzer DO")) -> ()
                n8000 = local write "System Status"("SEMI-AUTOMATIC MODE" ("System Status")) -> ()
                n8001 = local write "abort ch2"(FALSE) -> ()
              }
            }
            n8002 = case shown="True" w13600 {
              frame False {
              }
              frame True {
                n8003 = local write "CH2_TP_BV_DO"(FALSE ("Buzzer DO")) -> ()
              }
            }
            n8004 = case shown="True" w13609 {
              frame False {
              }
              frame True {
                w13623 = FALSE ("CH1_Trns_BP_Left_DO")
                w13625 = FALSE
                w13626 = FALSE
                w13624 = FALSE ("CH1_CC_DO")
                n8005 = local write "Buzzer DO"(TRUE ("Buzzer DO")) -> ()
                n8006 = local write "1-2 tr"(w13626) -> ()
                n8007 = local write "1-3 tr"(w13626) -> ()
                n8008 = local write "1-4 tr"(w13626) -> ()
                n8009 = local write "2-1 tr"(w13626) -> ()
                n8010 = local write "2-3 tr"(w13626) -> ()
                n8011 = local write "2-4 tr"(w13626) -> ()
                n8012 = local write "3-1 tr"(w13626) -> ()
                n8013 = local write "3-2 tr"(w13626) -> ()
                n8014 = local write "3-4 tr"(w13626) -> ()
                n8015 = local write "4-1 tr"(w13626) -> ()
                n8016 = local write "4-2 tr"(w13626) -> ()
                n8017 = local write "4-3 tr"(w13626) -> ()
                n8018 = local write "Casette_Servo_Start/Stop DO"(FALSE ("Casette_Servo_Start/Stop DO")) -> ()
                n8019 = local write "CH2_Trns_BP_Left_DO"(w13623) -> ()
                n8020 = local write "CH2_Trns_BP_Right_DO"(w13623) -> ()
                n8021 = local write "CH2_CC_DO"(w13624) -> ()
                n8022 = local write "ch2 pumpdown alg"(w13624) -> ()
                n8023 = local write "Pump Down CH2"(w13624) -> ()
                n8024 = local write "ch2 shutdown alg"(w13624) -> ()
                n8025 = local write "Shut Down CH2"(w13624) -> ()
                n8026 = local write "ch1-2 transfer"(w13625) -> ()
                n8027 = local write "ch2-3 transfer"(w13625) -> ()
                n8028 = local write "ch3-4 transfer"(w13625) -> ()
                n8029 = local write "ch2-1 transfer"(w13625) -> ()
                n8030 = local write "ch3-2 transfer"(w13625) -> ()
                n8031 = local write "ch4-3 transfer"(w13625) -> ()
              }
            }
            n8032 = case shown="True" w13603 {
              frame False {
              }
              frame True {
                w13619 = TRUE ("Buzzer DO")
                n8033 = local write "Tp2 auto stop"(w13619) -> ()
                n8034 = local write "pcgv2 auto close"(w13619) -> ()
                n8035 = local write "Dc_auto_off"(FALSE ("Dc_auto_off")) -> ()
                n8036 = local write "System Status"("CH2 ABORTED" ("System Status")) -> ()
              }
            }
            n8037 = case shown="True" w13596 {
              frame False {
              }
              frame True {
                n8038 = local write "CH2_PL_VBV_DO"(TRUE) -> ()
                n8039 = local write "CH2_MP_DO"(FALSE ("Buzzer DO")) -> ()
              }
            }
          }
        }
        n8040 = feedback-in #311(w13591) -> ()
      }
      frame #4 {
        # "argon \nflow off"
        n8041 = feedback #312() -> (w13667:bool)  [unwired: 1 in]
        n8042 = feedback #313() -> (w13664:bool)  [unwired: 1 in]
        n8043 = case shown="True" "abort ch4" {
          tunnel: w13667 -> [_ w13720]
          tunnel: [TRUE FALSE] -> w13666
          frame False {
          }
          frame True {
            n8044 = call "Elapsed Time152"("Auto Reset"=w13720) -> ("Elapsed Time (s)"=w13704:dbl)  [unwired: 11 in, 7 out]
            n8045 = In Range and Coerce(upper limit=5.5, x=w13704, lower limit=0.0) -> (In Range?=w13716:bool)  [unwired: 1 out]
            n8046 = In Range and Coerce(upper limit=1.5, x=w13704, lower limit=0.0) -> (In Range?=w13710:bool)  [unwired: 1 out]
            n8047 = In Range and Coerce(upper limit=9.5, x=w13704, lower limit=8.5) -> (In Range?=w13713:bool)  [unwired: 1 out]
            n8048 = In Range and Coerce(upper limit=8.0, x=w13704, lower limit=7.0) -> (In Range?=w13703:bool)  [unwired: 1 out]
            n8049 = In Range and Coerce(upper limit=6.5, x=w13704, lower limit=5.5) -> (In Range?=w13707:bool)  [unwired: 1 out]
            n8050 = case shown="True" w13713 {
              frame False {
              }
              frame True {
                n8051 = local write "Buzzer DO"(FALSE ("Buzzer DO")) -> ()
                n8052 = local write "System Status"("SEMI-AUTOMATIC MODE" ("System Status")) -> ()
                n8053 = local write "abort ch4"(FALSE ("Buzzer DO")) -> ()
              }
            }
            n8054 = case shown="True" w13707 {
              frame False {
              }
              frame True {
                n8055 = local write "CH4_TP_BV_DO"(FALSE ("Buzzer DO")) -> ()
              }
            }
            n8056 = case shown="True" w13716 {
              frame False {
              }
              frame True {
                w13731 = FALSE
                w13732 = FALSE
                w13729 = FALSE ("CH1_CC_DO")
                n8057 = local write "Buzzer DO"(TRUE ("Buzzer DO")) -> ()
                n8058 = local write "1-2 tr"(w13732) -> ()
                n8059 = local write "1-3 tr"(w13732) -> ()
                n8060 = local write "1-4 tr"(w13732) -> ()
                n8061 = local write "2-1 tr"(w13732) -> ()
                n8062 = local write "2-3 tr"(w13732) -> ()
                n8063 = local write "2-4 tr"(w13732) -> ()
                n8064 = local write "3-1 tr"(w13732) -> ()
                n8065 = local write "3-2 tr"(w13732) -> ()
                n8066 = local write "3-4 tr"(w13732) -> ()
                n8067 = local write "4-1 tr"(w13732) -> ()
                n8068 = local write "4-2 tr"(w13732) -> ()
                n8069 = local write "4-3 tr"(w13732) -> ()
                n8070 = local write "Casette_Servo_Start/Stop DO"(FALSE ("Casette_Servo_Start/Stop DO")) -> ()
                n8071 = local write "CH4_Trns_BP_Right_DO"(FALSE ("CH1_Trns_BP_Left_DO")) -> ()
                n8072 = local write "CH4_CC_DO"(w13729) -> ()
                n8073 = local write "ch4 pumpdown alg"(w13729) -> ()
                n8074 = local write "Pump Down CH4"(w13729) -> ()
                n8075 = local write "ch4 shutdown alg"(w13729) -> ()
                n8076 = local write "Shut Down CH4"(w13729) -> ()
                n8077 = local write "ch1-2 transfer"(w13731) -> ()
                n8078 = local write "ch2-3 transfer"(w13731) -> ()
                n8079 = local write "ch3-4 transfer"(w13731) -> ()
                n8080 = local write "ch2-1 transfer"(w13731) -> ()
                n8081 = local write "ch3-2 transfer"(w13731) -> ()
                n8082 = local write "ch4-3 transfer"(w13731) -> ()
              }
            }
            n8083 = case shown="True" w13710 {
              frame False {
              }
              frame True {
                w13725 = TRUE ("Buzzer DO")
                n8084 = local write "Tp4 auto stop"(w13725) -> ()
                n8085 = local write "pcgv4 auto close"(w13725) -> ()
                n8086 = local write "System Status"("CH4 ABORTED" ("System Status")) -> ()
              }
            }
            n8087 = case shown="True" w13703 {
              frame False {
              }
              frame True {
                n8088 = local write "CH4_PL_VBV_DO"(TRUE) -> ()
                n8089 = local write "CH4_MP_DO"(FALSE ("Buzzer DO")) -> ()
              }
            }
          }
        }
        n8090 = feedback-in #312(w13666) -> ()
        n8091 = case shown="True" "abort ch3" {
          tunnel: w13664 -> [_ w13686]
          tunnel: [TRUE FALSE] -> w13665
          frame False {
          }
          frame True {
            n8092 = call "Elapsed Time153"("Auto Reset"=w13686) -> ("Elapsed Time (s)"=w13670:dbl)  [unwired: 11 in, 7 out]
            n8093 = In Range and Coerce(upper limit=5.5, x=w13670, lower limit=0.0) -> (In Range?=w13682:bool)  [unwired: 1 out]
            n8094 = In Range and Coerce(upper limit=1.5, x=w13670, lower limit=0.0) -> (In Range?=w13676:bool)  [unwired: 1 out]
            n8095 = In Range and Coerce(upper limit=9.5, x=w13670, lower limit=8.5) -> (In Range?=w13679:bool)  [unwired: 1 out]
            n8096 = In Range and Coerce(upper limit=8.0, x=w13670, lower limit=7.0) -> (In Range?=w13669:bool)  [unwired: 1 out]
            n8097 = In Range and Coerce(upper limit=6.5, x=w13670, lower limit=5.5) -> (In Range?=w13673:bool)  [unwired: 1 out]
            n8098 = case shown="True" w13679 {
              frame False {
              }
              frame True {
                n8099 = local write "Buzzer DO"(FALSE ("Buzzer DO")) -> ()
                n8100 = local write "System Status"("SEMI-AUTOMATIC MODE" ("System Status")) -> ()
                n8101 = local write "abort ch3"(FALSE ("Buzzer DO")) -> ()
              }
            }
            n8102 = case shown="True" w13673 {
              frame False {
              }
              frame True {
                n8103 = local write "CH3_TP_BV_DO"(FALSE ("Buzzer DO")) -> ()
              }
            }
            n8104 = case shown="True" w13682 {
              frame False {